vi "UHR-Fleezers Control (host) - 10.2.vi"() -> ()   [LabVIEW 2009]
uses:
  <vilib>/Utility/miscctls.llb/LVPoint32TypeDef.ctl
  <vilib>/Utility/miscctls.llb/LVMinMaxIncTypeDef.ctl
  <vilib>/userDefined/High Color/nirio_resource_hc.ctl
  <vilib>/Instr/_visa.llb/VISA Configure Serial Port (Instr).vi
  <vilib>/Platform/TimedLoop/XDataNode/XDataNode.xnode
  <vilib>/Platform/TimedLoop/XDataNode/loadlvalarms.vi
  <vilib>/Platform/TimedLoop/XDataNode/timing_clust.ctl
  <vilib>/Platform/TimedLoop/XDataNode/nitl_modes.ctl
  <vilib>/Platform/TimedLoop/XDataNode/wakeup.ctl
  <vilib>/rvi/interface/nirviOpenFPGA/nirviOpenFPGA.xnode
  FPGA Bitfiles/UHR-Fleezers Instr~F0_FPGA Target_UHR-Fleezers Contr~5A.lvbitx
  UHR-Fleezers Control (fpga) - 10.3.vi
  <vilib>/FPGAPlugInAG/PCIe-7852R/nirviIntfOpen_PCIe-7852R.vi
  <vilib>/rvi/interface/nirviMethod/nirviMethod.xnode
  <vilib>/Utility/error.llb/Merge Errors.vi
  <vilib>/LabVIEW Targets/FPGA/Rio/nirio_HostInterface/nirio_Reset.vi
  <vilib>/LabVIEW Targets/FPGA/Rio/nirio_HostInterface/nirio_DMAStopAll.vi
  <vilib>/rvi/interface/common/niFpgaNodeNameForErrorReporting.ctl
  <vilib>/rvi/errors/niLvFpgaWhatHappensToTopLevelVI.ctl
  <vilib>/LabVIEW Targets/FPGA/Rio/nirio_HostInterface/nirio_DisableInterrupts.vi
  <vilib>/Utility/error.llb/Error Cluster From Error Code.vi
  <vilib>/rvi/errors/niLvFpgaAdjustHostInterfaceError.vi
  <vilib>/rvi/interface/nirviReadWriteControl/nirviReadWriteControl.xnode
  <vilib>/LabVIEW Targets/FPGA/Rio/nirio_HostInterface/nirio_WriteBig.vi
  <vilib>/LabVIEW Targets/FPGA/Rio/nirio_HostInterface/nirio_DMAConfigure.vi
  <vilib>/RVI Host/nirviSupport.llb/nirviErrorClusterFromErrorCode.vi
  <vilib>/LabVIEW Targets/FPGA/Rio/nirio_HostInterface/nirio_EnableInterrupts.vi
  <vilib>/rvi/errors/niLvFpgaReportInternalErrorWithAdditionalInfo.vi
  <vilib>/express/express analysis/Spectral/XNode/ExpressSpectralMeasurementsBlockNode.xnode
  <vilib>/express/express analysis/Spectral/Block/exnSpectralBlock spectral measurements PSD poly.vi
  <vilib>/express/express analysis/Spectral/Block/exnSpectralBlock spectral measurements PSD WFM.vi
  <vilib>/Waveform/WDTOps.llb/WDT Append Waveforms DBL.vi
  <vilib>/LabVIEW Targets/FPGA/Rio/nirio_HostInterface/nirio_ReadBig.vi
  <vilib>/rvi/interface/nirviCloseFPGA/nirviCloseFPGA.xnode
  FPGA Bitfiles/UHR-Fleezers Instr~3C_FPGA Target_UHR-Fleezers Contr~4B.lvbitx
  <vilib>/FPGAPlugInAG/PCIe-7852R/nirviIntfClose_PCIe-7852R.vi
  <vilib>/vision/Avi1.llb/AviRefnum.ctl
  <vilib>/Analysis/NI_AALBase.lvlib
  <vilib>/Platform/TimedLoop/XDataNode/XDNodeRunTimeDep.lvlib
  openfpgaref.8.6.ctl
  NiRioSrv.dll
  <vilib>/vision/NI_Vision_Development_Module.lvlib
panel:
  in  "Sample Channel Flow":bool=TRUE
  in  "Pump 3 contents":string="Left: ADig beads" caption="contents"
  in  "Pump 1 contents":string="Right: DNA beads" caption="contents"
  in  "Scripts":T1(tab)=enum."Tether Fishing"
  in  "Starting \nTrap Delta (MHz)":dbl=15.0
  in  "Take Force FB Data\nUpper Channel":bool
  in  "Cap 1 Samp Flow ON":bool
  in  "Cap 2 Samp Flow ON":bool=TRUE
  in  "Got DNA bead":bool
  in  "Got ADig bead":bool
  in  "Cap 2 Flow ON":bool=TRUE
  in  "Cap 1 Flow ON":bool=TRUE
  in  "Cap 2 T ON":bool=TRUE
  in  "Move Cap. 2 (ADig Left)":bool
  in  "Move Cap. 1 (DNA Right)":bool
  in  "Cal/Data Acq. Spot":bool
  in  "Dump Beads":bool
  in  "Lower Ch. Cap.":bool
  in  "Cap 1 T ON":bool=TRUE
  in  "Offset 2 Set":dbl=2.0
  in  "Offset 1 Set":dbl
  in  "Cal @ (MHz)":dbl=15.0
  in  "W/ Offset 1":bool=TRUE
  in  "Offset 1 Start (MHz)":dbl=13.0
  in  "W/ Offset 2":bool
  in  "Offset 2 Start (MHz)":dbl=16.0
  in  "Move to Delta 2 (MHz)":dbl=13.0
  in  "Attempt Limit":dbl=15.0 caption="Limit"
  out "Attempts":dbl=10.0
  in  "Wait Before Save (s)":u32=1
  in  "Fish for Tether":bool
  in  "Closest Delta (MHz)":dbl=9.25 step=0.25
  in  "Stop F (pN)":dbl=3.0
  in  "Then...":string(combo)="5"
  in  "Move to Delta 1 (MHz)":dbl=13.0
  in  "Tether Alarm?":bool=TRUE
  out "Tether":bool
  in  "TA Cancel Save?":bool
  in  "TA Green Off?":bool
  in  "Raster Set Upon Tether":u32=1
  in  "Save at end (5, 6)":bool
  in  "N Steps":dbl=20.0
  in  "Step Size (nm)":dbl=0.34
  in  "Save ave factor":dbl=1.0
  in  "Take Stepping Data":bool
  in  "Dip Trap Delta 1 (MHz)":dbl=15.0
  in  "Move Trap Before?":bool
  in  "Save Data After?":bool
  in  "Green ON After?":bool
  in  "Dip Trap Delta 2 (MHz)":dbl=15.0
  in  "Move Trap After?":bool
  in  "Duration (s)":dbl=1.0
  in  "Dip for Protein":bool
  in  "APD to Watch":bool
  out "Duration (s)":dbl
  in  "Action":string(combo)="Yank"
  in  "Fl. Triggered...":bool
  in  "Fl. Delta Thresh. (kHz)":dbl=0.6
  out "Waiting":bool
  out "Fl. High":bool
  in  "N pts to average":u16=6
  in  "Yank Delay (s)":dbl=3.5
  in  "Yank to Delta Array (MHz)":dbl[](array[numeric])=[16.3, 15.85, 14.85]
  in  "N Array El":u8=3 min=1 step=1
  in  "Random Choice":bool=TRUE
  in  "Force Yank":bool
  in  "Force Reset":bool
  in  "Y change (mm)":dbl
  in  "Profile":bool
  out "Current Position":cluster{dbl, dbl, dbl}
  out "Sigma/Mean 2":dbl=0.9156115002105881 caption="Sigma/Mean" format="%#_2g"
  out "Rate sigma (Hz) 2":dbl=91.25594618765528 caption="Sigma (Hz)" format="%0.2f"
  out "APD 2 Rate (Hz)":dbl=99.66666666666667 format="%#_3p"
  out "Primary Video Display":T2(plugin-control)
  out "Waveform Graph":dbl[](graph) caption="APD Line Scan"
  in  "Inject Pump 3":bool
  in  "Inject Pump 1":bool
  out "Messages":string="4:51 PM\tLost tether (7 s).\r4:51 PM\tFormed tether in 10 attempt(s).\r4:50 PM\tLost tether (5 s).\r4:49 PM\tFormed tether in 5 attempt(s).\r4:47 PM\tLost tether (36 s).\r4:47 PM\tFormed tether in 1 attempt(s).\r4:42 PM\tTether fishing timeout.\r4:37 PM\tTether fishing timeout.\r4:36 PM\tTether fishing timeout.\r4:32 PM\tTether fishing timeout.\r4:29 PM\tLost tether (4 s).\r4:28 PM\tFormed tether in 6 attempt(s).\r4:28 PM\tLost tether (5 s).\r4:28 PM\tFormed tether in 6 attempt(s).\r4:23 PM\tFormed tether in 1 attempt(s).\r4:23 PM\tLost tether (6 s).\r4:23 PM\tFormed tether in 1 attempt(s).\r4:14 PM\tFormed tether in 2 attempt(s).\r4:10 PM\tLost tether (548 s).\r4:01 PM\tFormed tether in 2 attempt(s).\r3:58 PM\tLost tether (6 s).\r3:58 PM\tFormed tether in 3 attempt(s).\r3:57 PM\tTether fishing timeout.\r3:42 PM\tLost tether (6 s).\r3:42 PM\tFormed tether in 6 attempt(s).\r3:39 PM\tLost tether (50 s).\r3:38 PM\tFormed tether in 10 attempt(s).\r3:37 PM\tLost tether (5 s).\r3:37 PM\tFormed tether in 6 attempt(s).\r3:34 PM\tTether fishing timeout.\r3:31 PM\tLost tether (45 s).\r3:30 PM\tFormed tether in 1 attempt(s).\r3:30 PM\tLost tether (4 s).\r3:30 PM\tFormed tether in 4 attempt(s).\r3:22 PM\tFormed tether in 6 attempt(s).\r3:18 PM\tLost tether (51 s).\r3:17 PM\tFormed tether in 3 attempt(s).\r3:17 PM\tLost tether (6 s).\r3:16 PM\tFormed tether in 1 attempt(s).\r3:06 PM\tFormed tether in 2 attempt(s).\r3:05 PM\tLost tether (3 s).\r3:05 PM\tFormed tether in 1 attempt(s).\r2:11 PM\tUHR-Fleezers ready.\r"
  in  "APD Ave N":dbl=10.0
  out "Int. Time (s)":dbl=3.0
  in  "Stop All":bool=TRUE
  out "Sigma/Mean":dbl=0.7461899027919234 format="%#_2g"
  out "Rate sigma (Hz)":dbl=246.24266792133471 caption="Sigma (Hz)" format="%0.2f"
  in  "Tab Control 6":T3(tab)
  in  "APD 2 Offset":dbl
  in  "APD 1 Offset":dbl
  out "RMS (Ang)":dbl=824.5898142565536 format="%_2g"
  in  "Bead Sep. Int. Time (s)":dbl=5.0 caption="Int. Time (s)"
  in  "Below (kHz)":dbl=0.5
  in  "Above (kHz)":dbl=2.0
  in  "Adjust Scale\nto Mean":bool
  in  "Rescale on Mean":bool
  in  "Offset (nm)":dbl
  out "Mean":dbl=107.85631162700733 caption="Mean (pN)" format="%#_3g"
  out "Force":waveform(dbl)[](graph)=[{"t0"=timestamp(9589.800000000116 s since 1904-01-01), "dt"=0.15, "Y"=[-107.59208218650274, -108.24679101361127], "attributes"=variant("NI_ChannelName"=variant(string "T1 X"))}, {"t0"=timestamp(9589.800000000116 s since 1904-01-01), "dt"=0.15, "Y"=[107.4628305657673, 108.12354274214799], "attributes"=variant("NI_ChannelName"=variant(string "T2 X"))}]
  out "APD Chart":waveform(dbl)[](graph)=[{"t0"=timestamp(9589.800000000116 s since 1904-01-01), "dt"=0.15, "Y"=[253.33333333333334, 266.6666666666667], "attributes"=variant("NI_ChannelName"=variant(string "APD 1"))}, {"t0"=timestamp(9589.800000000116 s since 1904-01-01), "dt"=0.15, "Y"=[93.33333333333334, 106.66666666666667], "attributes"=variant("NI_ChannelName"=variant(string "APD 2"))}]
  in  "Calibration":u16(ring)=2 items=["None", "Position", "Force"]
  out "T1 X":dbl=-107.919436600057 caption="T1 X (pN)" format="%0.2f"
  out "T2 X":dbl=-107.79318665395765 caption="T2 X (pN)" format="%0.2f"
  out "Bead Separation":waveform(dbl)(graph)={"t0"=timestamp(9589.800000000116 s since 1904-01-01), "dt"=0.15, "Y"=[-66.14062626515556, -66.57399525696837], "attributes"=variant("NI_ChannelName"=variant(string "T1 X"))}
  in  "Amplitude (nm)":dbl=3.0
  out "Bead Mean (nm)":dbl=-64.52066524805926 caption="Mean (nm)" format="%0.2f"
  out "Difference":dbl=0.12624994609934959 caption="Difference (pN)" format="%.2g"
  in  "Take Detection Laser\nImage":bool
  out "APD 2":T2(plugin-control) caption="APD 2 (Cy5)"
  in  "Flip Green Filter":bool
  in  "Set X Only":bool
  in  "Set Y Only":bool
  out "APD 1":T2(plugin-control) caption="APD 1 (Cy3)"
  out "Detection Laser Y":T2(plugin-control)
  out "Pointer Y (V)":dbl=4.98101801028038 format="%_3g"
  out "Pointer X (V)":dbl=3.881593676564837 format="%_3g"
  in  "Set Confocal Spot (X-Y)":bool
  out "Detection Laser X":T2(plugin-control)
  out "Saved APD":dbl[][](graph)=[[640.0, 640.0, 513.3333333333334, 520.0, 506.6666666666667, 520.0, 626.6666666666667, 680.0, 540.0, 606.6666666666667, 640.0, 513.3333333333334, 553.3333333333334, 693.3333333333334, 613.3333333333334, 513.3333333333334, 660.0, 513.3333333333334, 620.0, 506.6666666666667, 613.3333333333334, 546.6666666666667, 566.6666666666667, 753.3333333333334, 540.0, 546.6666666666667, 593.3333333333334, 646.6666666666667, 533.3333333333334, 613.3333333333334, 633.3333333333334, 653.3333333333334, 580.0, 646.6666666666667, 686.6666666666667, 660.0, 646.6666666666667, 560.0, 520.0, 600.0, 573.3333333333334, 633.3333333333334, 620.0, 600.0, 553.3333333333334, 533.3333333333334, 540.0, 546.6666666666667, 586.6666666666667, 573.3333333333334, 626.6666666666667, 506.6666666666667, 606.6666666666667, 613.3333333333334, 600.0, 526.6666666666667, 606.6666666666667, 606.6666666666667, 560.0, 613.3333333333334, 546.6666666666667, 486.6666666666667, 606.6666666666667, 573.3333333333334, 660.0, 693.3333333333334, 620.0, 586.6666666666667, 553.3333333333334, 506.6666666666667, 486.6666666666667, 593.3333333333334, 520.0, 560.0, 653.3333333333334, 633.3333333333334, 546.6666666666667, 653.3333333333334, 586.6666666666667, 566.6666666666667, 620.0, 546.6666666666667, 593.3333333333334, 580.0, 673.3333333333334, 673.3333333333334, 566.6666666666667, 620.0, 506.6666666666667, 633.3333333333334, 613.3333333333334, 546.6666666666667, 606.6666666666667, 600.0, 680.0, 586.6666666666667, 573.3333333333334, 540.0, 573.3333333333334, 633.3333333333334, 546.6666666666667, 553.3333333333334, 533.3333333333334, 633.3333333333334, 633.3333333333334, 600.0, 646.6666666666667, 640.0, 540.0, 486.6666666666667, 586.6666666666667, 566.6666666666667, 626.6666666666667, 606.6666666666667, 640.0, 546.6666666666667, 566.6666666666667, 653.3333333333334, 626.6666666666667, 586.6666666666667, 613.3333333333334, 626.6666666666667, 560.0, 700.0, 546.6666666666667, 506.6666666666667, 566.6666666666667, 640.0, 573.3333333333334, 593.3333333333334, 493.33333333333337, 613.3333333333334, 626.6666666666667, 673.3333333333334, 580.0, 633.3333333333334, 633.3333333333334, 713.3333333333334, 400.0, 560.0, 520.0, 506.6666666666667, 720.0, 553.3333333333334, 553.3333333333334, 426.6666666666667, 600.0, 540.0, 520.0, 640.0, 453.33333333333337, 533.3333333333334, 460.0, 426.6666666666667, 546.6666666666667, 580.0, 460.0, 480.0, 586.6666666666667, 473.33333333333337, 580.0, 613.3333333333334, 546.6666666666667, 500.0, 546.6666666666667, 540.0, 586.6666666666667, 560.0, 406.6666666666667, 533.3333333333334, 520.0, 573.3333333333334, 540.0, 486.6666666666667, 633.3333333333334, 486.6666666666667, 586.6666666666667, 440.0, 446.6666666666667, 553.3333333333334, 520.0, 540.0, 620.0, 506.6666666666667, 580.0, 653.3333333333334, 540.0, 566.6666666666667, 586.6666666666667, 453.33333333333337, 653.3333333333334, 553.3333333333334, 460.0, 593.3333333333334, 420.0, 553.3333333333334, 526.6666666666667, 480.0, 520.0, 606.6666666666667, 493.33333333333337, 560.0, 513.3333333333334, 426.6666666666667, 440.0, 513.3333333333334, 500.0, 633.3333333333334, 513.3333333333334, 460.0, 526.6666666666667, 466.6666666666667, 540.0, 546.6666666666667, 540.0, 486.6666666666667, 500.0, 506.6666666666667, 553.3333333333334, 400.0, 493.33333333333337, 420.0, 413.33333333333337, 540.0, 513.3333333333334, 493.33333333333337, 420.0, 533.3333333333334, 466.6666666666667, 546.6666666666667, 493.33333333333337, 480.0, 366.6666666666667, 526.6666666666667, 520.0, 406.6666666666667, 526.6666666666667, 620.0, 520.0, 500.0, 460.0, 480.0, 520.0, 446.6666666666667, 680.0, 526.6666666666667, 613.3333333333334, 700.0, 566.6666666666667, 646.6666666666667, 573.3333333333334, 593.3333333333334, 626.6666666666667, 546.6666666666667, 526.6666666666667, 773.3333333333334, 626.6666666666667, 546.6666666666667, 633.3333333333334, 553.3333333333334, 613.3333333333334, 546.6666666666667, 540.0, 593.3333333333334, 620.0, 646.6666666666667, 706.6666666666667, 506.6666666666667, 573.3333333333334, 640.0, 513.3333333333334, 473.33333333333337, 606.6666666666667, 533.3333333333334, 466.6666666666667, 506.6666666666667, 500.0, 573.3333333333334, 446.6666666666667, 646.6666666666667, 533.3333333333334, 533.3333333333334, 560.0, 500.0, 586.6666666666667, 580.0, 460.0, 486.6666666666667, 580.0, 573.3333333333334, 506.6666666666667, 533.3333333333334, 586.6666666666667, 700.0, 486.6666666666667, 480.0, 560.0, 593.3333333333334, 573.3333333333334, 680.0, 626.6666666666667, 633.3333333333334, 660.0, 640.0, 600.0, 600.0, 586.6666666666667, 760.0, 686.6666666666667, 613.3333333333334, 686.6666666666667, 593.3333333333334, 553.3333333333334, 606.6666666666667, 573.3333333333334, 460.0, 546.6666666666667, 640.0, 553.3333333333334, 600.0, 580.0, 526.6666666666667, 620.0, 573.3333333333334, 626.6666666666667, 506.6666666666667, 573.3333333333334, 413.33333333333337, 373.33333333333337, 493.33333333333337, 546.6666666666667, 513.3333333333334, 466.6666666666667, 626.6666666666667, 526.6666666666667, 486.6666666666667, 480.0, 500.0, 593.3333333333334, 453.33333333333337, 500.0, 460.0, 593.3333333333334, 540.0, 500.0, 486.6666666666667, 500.0, 533.3333333333334, 460.0, 540.0, 500.0, 580.0, 480.0, 586.6666666666667, 560.0, 513.3333333333334, 566.6666666666667, 553.3333333333334, 540.0, 593.3333333333334, 533.3333333333334, 493.33333333333337, 553.3333333333334, 466.6666666666667, 500.0, 646.6666666666667, 513.3333333333334, 540.0, 446.6666666666667, 540.0, 426.6666666666667, 540.0, 613.3333333333334, 506.6666666666667, 493.33333333333337, 486.6666666666667, 606.6666666666667, 500.0, 486.6666666666667, 526.6666666666667, 560.0, 540.0, 433.33333333333337, 540.0, 520.0, 480.0, 540.0, 473.33333333333337, 466.6666666666667, 420.0, 413.33333333333337, 560.0, 546.6666666666667, 493.33333333333337, 406.6666666666667, 480.0, 480.0, 466.6666666666667, 426.6666666666667, 486.6666666666667, 520.0, 606.6666666666667, 480.0, 493.33333333333337, 626.6666666666667, 486.6666666666667, 486.6666666666667, 440.0, 660.0, 593.3333333333334, 533.3333333333334, 520.0, 580.0, 500.0, 573.3333333333334, 500.0, 573.3333333333334, 446.6666666666667, 586.6666666666667, 586.6666666666667, 546.6666666666667, 600.0, 620.0, 540.0], [73.33333333333334, 166.66666666666669, 86.66666666666667, 113.33333333333334, 140.0, 126.66666666666667, 93.33333333333334, 93.33333333333334, 113.33333333333334, 120.0, 120.0, 146.66666666666669, 66.66666666666667, 113.33333333333334, 120.0, 113.33333333333334, 120.0, 126.66666666666667, 140.0, 133.33333333333334, 120.0, 140.0, 86.66666666666667, 160.0, 126.66666666666667, 113.33333333333334, 93.33333333333334, 133.33333333333334, 100.0, 126.66666666666667, 133.33333333333334, 86.66666666666667, 126.66666666666667, 80.0, 140.0, 113.33333333333334, 120.0, 186.66666666666669, 113.33333333333334, 93.33333333333334, 53.333333333333336, 66.66666666666667, 133.33333333333334, 140.0, 126.66666666666667, 53.333333333333336, 126.66666666666667, 133.33333333333334, 73.33333333333334, 113.33333333333334, 100.0, 66.66666666666667, 113.33333333333334, 120.0, 140.0, 100.0, 80.0, 126.66666666666667, 126.66666666666667, 133.33333333333334, 73.33333333333334, 113.33333333333334, 93.33333333333334, 126.66666666666667, 140.0, 46.66666666666667, 153.33333333333334, 113.33333333333334, 66.66666666666667, 106.66666666666667, 146.66666666666669, 100.0, 120.0, 93.33333333333334, 140.0, 126.66666666666667, 93.33333333333334, 60.0, 46.66666666666667, 133.33333333333334, 93.33333333333334, 113.33333333333334, 80.0, 73.33333333333334, 113.33333333333334, 93.33333333333334, 113.33333333333334, 146.66666666666669, 120.0, 66.66666666666667, 120.0, 106.66666666666667, 80.0, 113.33333333333334, 113.33333333333334, 100.0, 73.33333333333334, 106.66666666666667, 126.66666666666667, 80.0, 140.0, 93.33333333333334, 120.0, 113.33333333333334, 80.0, 53.333333333333336, 113.33333333333334, 80.0, 93.33333333333334, 140.0, 146.66666666666669, 93.33333333333334, 180.0, 133.33333333333334, 60.0, 140.0, 100.0, 153.33333333333334, 100.0, 86.66666666666667, 93.33333333333334, 106.66666666666667, 126.66666666666667, 60.0, 113.33333333333334, 153.33333333333334, 120.0, 140.0, 106.66666666666667, 86.66666666666667, 146.66666666666669, 113.33333333333334, 133.33333333333334, 126.66666666666667, 100.0, 126.66666666666667, 186.66666666666669, 86.66666666666667, 146.66666666666669, 73.33333333333334, 160.0, 113.33333333333334, 113.33333333333334, 80.0, 106.66666666666667, 126.66666666666667, 113.33333333333334, 93.33333333333334, 126.66666666666667, 126.66666666666667, 113.33333333333334, 93.33333333333334, 60.0, 146.66666666666669, 100.0, 106.66666666666667, 66.66666666666667, 80.0, 106.66666666666667, 93.33333333333334, 73.33333333333334, 113.33333333333334, 100.0, 86.66666666666667, 133.33333333333334, 100.0, 86.66666666666667, 100.0, 53.333333333333336, 180.0, 120.0, 133.33333333333334, 106.66666666666667, 80.0, 133.33333333333334, 86.66666666666667, 73.33333333333334, 100.0, 100.0, 126.66666666666667, 93.33333333333334, 73.33333333333334, 66.66666666666667, 113.33333333333334, 73.33333333333334, 140.0, 120.0, 133.33333333333334, 100.0, 86.66666666666667, 53.333333333333336, 100.0, 80.0, 100.0, 86.66666666666667, 106.66666666666667, 120.0, 73.33333333333334, 120.0, 60.0, 100.0, 113.33333333333334, 93.33333333333334, 126.66666666666667, 80.0, 73.33333333333334, 73.33333333333334, 100.0, 86.66666666666667, 66.66666666666667, 133.33333333333334, 93.33333333333334, 73.33333333333334, 126.66666666666667, 73.33333333333334, 106.66666666666667, 86.66666666666667, 120.0, 133.33333333333334, 80.0, 146.66666666666669, 80.0, 120.0, 86.66666666666667, 80.0, 60.0, 100.0, 93.33333333333334, 73.33333333333334, 106.66666666666667, 126.66666666666667, 80.0, 133.33333333333334, 86.66666666666667, 106.66666666666667, 120.0, 60.0, 40.0, 66.66666666666667, 86.66666666666667, 93.33333333333334, 66.66666666666667, 86.66666666666667, 100.0, 86.66666666666667, 120.0, 146.66666666666669, 80.0, 80.0, 160.0, 133.33333333333334, 93.33333333333334, 80.0, 140.0, 40.0, 113.33333333333334, 113.33333333333334, 93.33333333333334, 100.0, 106.66666666666667, 93.33333333333334, 133.33333333333334, 120.0, 120.0, 86.66666666666667, 66.66666666666667, 113.33333333333334, 66.66666666666667, 106.66666666666667, 100.0, 146.66666666666669, 120.0, 126.66666666666667, 106.66666666666667, 80.0, 133.33333333333334, 166.66666666666669, 86.66666666666667, 100.0, 133.33333333333334, 120.0, 86.66666666666667, 113.33333333333334, 40.0, 100.0, 106.66666666666667, 93.33333333333334, 86.66666666666667, 126.66666666666667, 53.333333333333336, 106.66666666666667, 106.66666666666667, 93.33333333333334, 80.0, 80.0, 120.0, 86.66666666666667, 146.66666666666669, 53.333333333333336, 86.66666666666667, 160.0, 153.33333333333334, 93.33333333333334, 93.33333333333334, 86.66666666666667, 120.0, 113.33333333333334, 93.33333333333334, 73.33333333333334, 60.0, 153.33333333333334, 60.0, 100.0, 80.0, 113.33333333333334, 106.66666666666667, 86.66666666666667, 113.33333333333334, 100.0, 86.66666666666667, 73.33333333333334, 100.0, 73.33333333333334, 80.0, 106.66666666666667, 93.33333333333334, 106.66666666666667, 106.66666666666667, 86.66666666666667, 60.0, 73.33333333333334, 93.33333333333334, 120.0, 140.0, 160.0, 60.0, 120.0, 120.0, 73.33333333333334, 73.33333333333334, 146.66666666666669, 80.0, 66.66666666666667, 100.0, 73.33333333333334, 113.33333333333334, 100.0, 66.66666666666667, 66.66666666666667, 93.33333333333334, 73.33333333333334, 146.66666666666669, 120.0, 86.66666666666667, 60.0, 86.66666666666667, 113.33333333333334, 120.0, 120.0, 73.33333333333334, 153.33333333333334, 106.66666666666667, 100.0, 80.0, 86.66666666666667, 113.33333333333334, 73.33333333333334, 113.33333333333334, 140.0, 93.33333333333334, 93.33333333333334, 60.0, 126.66666666666667, 93.33333333333334, 106.66666666666667, 113.33333333333334, 46.66666666666667, 113.33333333333334, 86.66666666666667, 100.0, 126.66666666666667, 93.33333333333334, 66.66666666666667, 160.0, 146.66666666666669, 93.33333333333334, 93.33333333333334, 93.33333333333334, 73.33333333333334, 106.66666666666667, 86.66666666666667, 66.66666666666667, 80.0, 86.66666666666667, 100.0, 120.0, 80.0, 120.0, 120.0, 133.33333333333334, 86.66666666666667, 113.33333333333334, 160.0, 93.33333333333334, 86.66666666666667, 93.33333333333334, 80.0, 120.0, 73.33333333333334, 93.33333333333334, 73.33333333333334, 73.33333333333334, 66.66666666666667, 120.0, 93.33333333333334, 60.0, 100.0, 100.0, 73.33333333333334, 73.33333333333334, 106.66666666666667, 86.66666666666667, 66.66666666666667, 126.66666666666667]] caption="Most Recent Time Trace"
  out "Trap Delta Graph":dbl[](graph)=[-106.43043807216529, -106.5454367986324, -106.51686160160939, -106.58501313534859, -106.73405579848394, -106.59345831600089, -106.55808478718131, -106.54847798904014, -106.63246708958809, -106.64841693959238, -106.4822053501463, -106.57755688373177, -106.67016724634344, -106.45433878652537, -106.47815911583766, -106.42379428925383, -106.51151845331754, -106.68746141834603, -106.50723577160747, -106.41173347001666, -106.45298074469062, -106.68357946354386, -106.41957394891901, -106.42779113376133, -106.46017439309665, -106.3331576187891, -106.35502678934324, -106.32337366489861, -106.55680288846125, -106.29647485921345, -106.4777976983645, -106.297812998571, -106.39808607771205, -106.65261139520646, -106.51296579380772, -106.66918631936434, -106.17562143548844, -84.60994919536043, 1.3310857319345684, 1.0361871672274952, 0.6560712621147459, 0.5689432704114208, 0.5054763131013246, 0.026676923553220266, 0.4416019568801436, 0.2735431213660061, 0.23024753352250904, 0.37724536348759063, 0.2421264893459717, 0.26340021780432943, 0.29841957537993546, 0.17548186500256102, 0.14535336814513755, 0.07167026524356301, 0.22596132502466781, 0.2852071568323358, 0.3257436622559723, 0.12892633791448793, 0.17014124062038827, 0.13608261272222044, 0.2165257310266071, 0.02390519326463647, 0.24374284074938912, 0.14033144222620686, 0.20160694442302618, 0.24399108515159418, 0.37280924880476496, 0.39269031828135303, 0.0020045770407064456, 0.24243253128233844, 0.5509136378777598, -0.06739948998052048, 0.3753325270901159, 0.041556923442069515, 0.5156644188755136, 0.43429902173750445, 0.6734298753615677, 0.24078809415362, 0.2226386778369127, 0.0928074556229388, 0.23452704613553288, 0.29537252172755735, 0.24028041004987544, 0.5110751644361885, 0.3115531148109213, 0.3541005104538466, 0.19808764601755413, 0.29451725645941296, 0.37483027387224876, 0.14422108697133207, 0.10937006932469684, -0.10006183935749324, 0.5174008122551468, -0.15899440920889152, 0.067222901985028, 0.4893964012215861, 0.16100705380999392, 0.040244638366899954, 0.21823030270568278, 0.2724552172281144, 0.3286154371444875, 0.09671105698981519, 0.211070673931971, 0.27403940383827663, -0.18158626168544867, 0.359992544087572, 0.17521597973752523, -0.01712139810390334, 0.34828383230753013, 0.38821465356197205, -0.47577316993658636, -0.061209978340928006, -0.04336067966990298, 0.1973437946223825, 0.14125329725782476, 0.39799396471853143, 0.5095924157430234, 0.5369250733859182, 0.5141657617439718, 0.12314529776262206, 0.12340359436175818, 0.4247246292008219, 0.34987918195615864, 0.3691260807314214, 0.18948963934016738, 0.11514675643557093, 0.3145960367967432, 0.0847238153799148, 0.5498257841297541, 0.3435810561376562, 0.28951709031660544, 0.11486034175086168, 0.19981958245548992, 0.24902605730103988, 0.08386197607169354, 0.3076486879407194, 0.5316368497813708, 0.011172428028344061, 0.16515294490283083, 0.2589832302335102, 0.06118106222967257, 0.05179602677324213, 0.14605031191417106, -0.27028691855927245, 0.3046427258477053, -0.32654161566760187, 0.11547372002670883, 0.05841771855848377, -0.09021888308668857, 0.28492200832706416, 0.14848195262761732, 0.08004379230789829, 0.11340489372509398, -0.1207310131639201, 0.1541946406564236, 0.1269929332462834, -0.25254475570349794, 0.1559630190503728, -0.16465543631295051, 0.11133039420408519, 0.1402543807831096, 0.02125799385333696, -0.16462459978957333, -0.38923305887864584, -0.02381113492727646, 0.10391530706475595, 0.23820889685935479, -0.023728686724600878, -0.04764111901766144, -0.007608743009235641, -0.2831431266449582, -0.4601669034291135, 0.1270783916843988, 0.11151315228001513, 0.07486139973609482, -0.24727183052659096, 0.19791921503036844, 0.07911640381694093, -0.06594038816975148, 0.2904115238995478, 0.2572744514721885, -0.20695214319298796, -0.011134088990943897, -0.1329170956283653, -0.17359323758311615, 0.12181978652209512, -0.11042971273973787, 0.22899157117508717, 0.3140832953715535, -0.30689327909618325, 0.03860844834068772, 0.394228107655571, 0.05293892569083136, -0.25365611830805873, 0.24686577579815186, 0.049501080171641065, -0.14974810230810087, -0.02833685388093199, 0.18652778365699527, 0.29108264069094064, -0.0008448102460272833, 0.0018380106327957058, 0.12078335855310426, 0.25940308098841486, -0.04482483301124446, 0.07376288462566721, -0.20968097306502337, -0.21601485851555285, -0.255227346307366, -0.006578989879893332, 0.2693875220630272, -0.05322628288934911, 0.013224520397867853, 0.019089251473903474, 0.1785683517670636, 0.0005106496658305038, 0.03471794306860293, -0.03881457062500418, 0.1314922052228636, 0.19291503243930383, 0.016286528257771483, 0.04613488933487331, 0.023391462208254027, -0.0867936685376553, 0.1667056535330356, 0.13551569687601753, 0.03966388491544098, -0.001509757708971271, -0.04930535048489537, -0.02488348604948106, 0.17699798141823225, 0.09067749598174343, 0.2810609960550859, -0.17953434343886976, -0.08087810161787876, 0.15531385466958078, 0.07966370440497603, 0.21169243968790535, 0.27463644895840034, 0.11358419137524867, 0.44151340468279066, 0.013676594736444725, 0.13803367875581318, 0.16762306170228025, -9.305097846396249, -8.734185730622158, -7.795085141730819, -7.1169239424821455, -6.8078194604182505, -6.012872438821646, -5.297070121155155, -4.8008820282039935, -3.80266145736694, -3.2398214424229104, -2.6995113604562464, -2.250937951595689, -1.6142815413389022, -1.1477956359922619, -0.7851258896920497, -0.5489468717661414, 0.007892963192939528, 0.4297874535410666, 0.7232126615705075, 1.0881378793787722, 0.9469945823546175, 1.1315981032380298, 1.5088200228939004, 1.9696025136662745, 2.0125320503247393, 2.0616893854058578, 2.0607414539584012, 2.6901101639116844, 2.913370534266508, 2.9915343321096253, 3.1810584698757345, 3.2694738112071233, 3.815351721905264, 3.711465789182815, 3.3319100390246166, 3.4738940838355026, 2.9938700615022165, 2.8719830063163836, 2.814001855577777, 2.4799945954145404, 2.306309702543458, 2.287683746001849, 1.884452351748454, 1.4763570637661683, 1.500909948307402, 1.3757091991201318, 0.9511484877404002, 0.7750514269276616, 0.6476631465563494, -0.070662296735875, -0.029594788212394696, -0.32400306754623637, -0.8864635561709634, -1.4877222685335405, -2.0507065584317017, -2.6968184066815972, -3.0471461188113667, -3.5358182192812335, -4.376697785171516, -4.953120166587164, -5.848565647315136, -6.053854911411889, -7.052139284154087, -7.172726882840011, -8.190341884763662, -8.57176218146154, -9.031969641304759, -9.160140089904607, -19.406396896392515, -20.72767491143481, -22.52957503831575, -24.628780001646625, -27.645919716135815, -31.524820294981247, -36.00375847806328, -40.29138452034995, -45.564980244900866, -52.03629009220346, -59.389338493635734, -67.53729872875331, -76.40368321454261, -86.00318733592643, -95.67183386111026, -98.591914485014, -103.5540396015088, -111.71602156262952, -119.7345182693686, -128.10083921857876, -133.92328842606133, -140.30486296175064, -152.13782681810846, -127.59977417259103, 1.9097381969808318, 2.146077316363836, 2.5695963953157115, 2.6372377874037967, 2.712002965976897, 2.21214115543342, 2.0827027656517636, 1.7918328994151387, 1.8334538504789635, 1.4887474407240884, 1.3183156469574928, 1.1074607806068812, 0.5449613088181862, 0.6411310292885716, 0.2865682674798876, -0.20561912550425498, -0.4283737772873612, -0.8213909015749081, -1.301367318197441, -1.4043123386109424, -2.455428847708026, -2.865387975996997, -3.4460393734956574, -4.088620933822033, -4.852423708406629, -5.363424054600309, -5.985200931385475, -6.449778687075328, -7.359018465262011, -8.014348652381976, -8.602206142039282, -9.11747831938223, -16.10276890966618, -16.652936161554457, -17.45363480985382, -18.573158822709363, -19.611725824538883, -21.567924207070938, -24.090533940752877, -27.20500645507802, -31.47067005386945, -36.72043318743074, -43.01369354998713, -50.30269462184975, -58.470394481182154, -66.68608952303441, -76.32223565208024, -85.90747526669313, -96.45584392830432, -107.64327334791787, -118.00360649269274, -128.23147312175695, -139.24390140541698, -150.1280581951645, -160.43369113902202, -169.03532569855338, -179.6526957081072, -190.15619730232487, -196.645730104612, -206.28355442560365, -205.5533003536683, -193.35735124448496, -181.88474031887915, -171.53558469680792, -161.06805576546705, -150.48071337332783, -140.05252361639847, -129.1694172743015, -118.51016094139078, -38.66402558537719, 0.4687738479286786, -0.017898865181683668, -0.38393700946650355, -0.7924297107116016, -1.2685508455729173, -1.7227958503540475, -2.5497829209829965, -3.131493827362692, -3.3162470336029233, -4.01435852437743, -4.494030889765619, -5.58945592615083, -6.219129572016236, -6.884133384184377, -7.124206108411009, -8.080705713244733, -8.622535042543017, -9.408401169796818] caption="Most Recent Time Trace"
  out "Save APD Deriv":dbl[][](graph)=[[0.0, 0.0, 0.0, 4.444444444444457, 23.33333333333337, 44.44444444444446, 30.0, 7.777777777777828, -10.0, -20.0, -11.111111111111086, 10.000000000000114, 23.33333333333337, 31.111111111111086, -22.222222222222285, 17.77777777777783, 2.2222222222221717, 64.44444444444446, 17.777777777777715, 2.2222222222222854, -54.44444444444446, -38.888888888888914, -26.666666666666742, -23.33333333333337, -35.55555555555543, -22.22222222222217, 20.000000000000114, 24.444444444444343, 30.0, 0.0, -10.0, -28.888888888888914, 8.8888888888888, 53.33333333333337, 38.888888888888914, -36.66666666666663, -86.66666666666663, -28.888888888888914, 36.66666666666663, 70.0, 12.222222222222285, -12.222222222222172, 7.777777777777715, 31.111111111111086, 30.0, -33.33333333333326, -33.33333333333337, -6.666666666666629, 16.66666666666663, 13.333333333333371, -35.55555555555566, -18.888888888888914, -14.444444444444457, 44.44444444444446, 12.222222222222172, -5.555555555555543, -45.55555555555554, 4.444444444444571, 28.888888888888914, 34.44444444444446, 16.66666666666663, 12.222222222222172, -11.111111111111086, -25.555555555555543, -47.777777777777715, -12.222222222222285, 8.888888888888914, 32.22222222222217, 63.33333333333337, -8.888888888888914, -47.77777777777783, -100.0, -40.0, 10.0, 3.3333333333332575, 1.1111111111110858, -60.0, -46.66666666666663, -55.5555555555556, 15.555555555555543, 32.222222222222285, 57.77777777777777, 33.33333333333337, 14.444444444444457, -21.111111111111086, -24.444444444444457, -36.66666666666674, 11.111111111111086, -1.1111111111110858, 14.444444444444457, -25.555555555555543, 2.2222222222221717, 45.55555555555554, 63.33333333333337, 32.222222222222285, -11.111111111111086, -27.77777777777783, -24.444444444444457, -53.333333333333314, -32.22222222222217, -7.777777777777828, 14.4444444444444, -26.666666666666686, -26.66666666666663, -10.0, 25.5555555555556, 4.444444444444457, 7.777777777777828, 3.3333333333332575, -11.111111111111143, -38.888888888888914, -50.0, -18.888888888888857, 6.666666666666686, 25.5555555555556, 11.111111111111086, -5.555555555555543, -30.0, 4.444444444444457, 35.555555555555486, 52.22222222222223, -6.666666666666686, 3.3333333333333712, 63.33333333333326, 134.4444444444445, 96.66666666666674, 11.1111111111112, -15.555555555555543, -7.777777777777828, 17.777777777777715, -20.0, -27.77777777777783, -16.66666666666663, 15.555555555555543, 35.55555555555554, -24.444444444444457, -45.55555555555554, -98.8888888888888, -37.77777777777783, -33.33333333333337, 22.22222222222217, 5.555555555555657, 25.555555555555543, -10.0, 7.777777777777715, -25.555555555555543, 51.111111111111086, 4.444444444444457, 44.44444444444446, -17.777777777777715, 62.22222222222217, 67.77777777777771, 64.44444444444446, 30.0, 5.555555555555543, 27.777777777777715, -17.777777777777715, -62.22222222222217, -91.11111111111109, -61.111111111111086, -4.444444444444457, 12.222222222222172, 10.0, -22.22222222222217, -77.77777777777771, -86.66666666666669, -48.888888888888914, 30.0, 28.888888888888857, 3.3333333333333144, -30.000000000000057, 8.888888888888914, 6.666666666666686, 27.77777777777777, -20.0, 5.555555555555543, -1.1111111111110858, 33.33333333333337, 24.444444444444457, 30.0, 10.0, -13.333333333333371, -22.22222222222217, -10.0, 1.1111111111110858, -31.111111111111143, -24.444444444444457, -19.999999999999943, 33.333333333333314, 4.444444444444457, 25.5555555555556, -20.0, -4.444444444444571, -38.88888888888897, -31.111111111111086, -33.33333333333326, -14.4444444444444, 0.0, 0.0, -25.5555555555556, 14.444444444444457, 23.333333333333314, 77.77777777777777, 4.4444444444444, 46.666666666666686, 3.3333333333333712, 62.22222222222223, -14.444444444444457, -10.0, -20.0, 22.222222222222285, 51.111111111111086], [0.0, 0.0, 0.0, -8.888888888888886, -3.3333333333333286, -3.3333333333333286, 4.444444444444443, -1.1111111111111143, -4.444444444444457, 12.222222222222214, 16.666666666666657, 20.0, -1.1111111111111143, -11.1111111111111, -14.444444444444443, -12.222222222222214, -10.000000000000014, -2.2222222222222143, 15.555555555555557, 18.8888888888889, -7.777777777777786, -27.777777777777786, -32.22222222222223, 13.333333333333343, 4.444444444444457, 6.666666666666671, -21.111111111111114, 2.2222222222222143, 11.111111111111114, 20.0, 2.2222222222222285, -2.2222222222222285, -18.888888888888886, 3.3333333333333286, -6.666666666666657, 15.555555555555557, -6.666666666666671, 16.666666666666657, -8.8888888888889, -5.555555555555557, -31.111111111111114, -15.555555555555557, -5.555555555555543, 13.333333333333343, 18.8888888888889, 17.77777777777777, -2.2222222222222285, -3.333333333333343, -14.444444444444443, -1.1111111111111143, -2.2222222222222143, 14.444444444444443, 0.0, -10.0, -18.888888888888886, 11.111111111111114, 37.77777777777777, 32.222222222222214, 16.66666666666667, -24.444444444444443, -18.888888888888886, -32.22222222222223, 2.2222222222222285, 12.222222222222214, 24.444444444444443, 10.0, 1.4210854715202004e-14, 4.444444444444457, 7.7777777777777715, 1.1111111111111143, 3.3333333333333286, -12.222222222222214, -3.333333333333343, -22.22222222222223, 1.1111111111111, -5.555555555555557, 5.555555555555557, -12.222222222222214, -17.77777777777777, -18.888888888888886, -14.444444444444443, 2.2222222222222143, 8.888888888888886, 12.222222222222214, 13.333333333333329, 11.111111111111114, 11.111111111111114, 1.1111111111111143, -15.555555555555557, -8.888888888888886, -15.555555555555543, -1.1111111111111143, -10.0, 13.333333333333329, 13.333333333333329, 5.555555555555543, -21.111111111111114, -21.1111111111111, -4.444444444444443, 7.7777777777777715, 10.0, 7.777777777777786, 3.333333333333343, -6.666666666666671, -22.22222222222223, -5.555555555555557, 5.555555555555557, 21.111111111111114, 5.555555555555557, 3.3333333333333286, 6.666666666666671, 10.0, -4.444444444444443, -17.777777777777786, -22.22222222222223, 1.1111111111111143, 11.111111111111114, 23.33333333333333, -5.555555555555557, -21.111111111111114, -40.0, -7.7777777777777715, 12.222222222222229, 34.44444444444446, 28.888888888888886, 23.33333333333333, 11.1111111111111, -12.222222222222229, -18.888888888888886, -19.999999999999986, 6.666666666666671, 15.555555555555557, 8.888888888888886, -11.111111111111114, -22.22222222222223, 5.555555555555557, 22.22222222222223, 28.8888888888889, 7.7777777777777715, -1.1111111111111143, -3.333333333333343, -17.777777777777786, -22.22222222222223, -25.555555555555557, -4.444444444444443, 1.1111111111111143, 4.444444444444443, 3.333333333333343, 5.555555555555557, 1.1111111111111143, 16.66666666666667, 5.555555555555557, 22.22222222222223, -14.444444444444457, -15.555555555555557, -25.555555555555557, -12.222222222222214, 11.111111111111114, 7.7777777777777715, 13.333333333333329, -8.888888888888886, -14.444444444444443, -13.333333333333329, 1.1111111111111143, 7.777777777777786, 0.0, 1.1111111111111, 14.444444444444443, 32.222222222222214, 5.555555555555557, -5.555555555555557, -30.0, -4.444444444444443, -15.555555555555557, -4.444444444444443, -5.555555555555557, 11.111111111111114, 10.0, 6.666666666666671, -2.2222222222222285, 18.8888888888889, 7.7777777777777715, 11.111111111111114, -20.0, -2.2222222222222143, -11.111111111111114, 6.666666666666657, -4.444444444444443, 4.444444444444443, -6.666666666666657, -4.444444444444443, 5.555555555555557, 20.0, 14.444444444444443, -4.444444444444443, -27.777777777777786, -25.555555555555557, -11.111111111111114, 11.1111111111111, 28.888888888888886, 18.888888888888886, 20.000000000000014, -6.666666666666671, -3.3333333333333286, -26.66666666666667, -20.0, -22.222222222222214, -10.0, 4.444444444444443, 0.0, 8.888888888888886, -1.1111111111111]] caption="Most Recent Time Trace"
  out "Delta Fl. 1":dbl=51.111111111111086
  out "Delta Fl. 2":dbl=-1.1111111111111